vi "HFRR ADV v042.vi"() -> ()   [LabVIEW 2025] (continued)
            n2226 = call-poly <vilib>:"Mean.vi"("X"=w2445) -> ("mean"=→"КОФ2 4":dbl)  [unwired: 1 out]
            n2227 = call-poly <vilib>:"Mean.vi"("X"=w2508) -> ("mean"=→"КОФ3":dbl)  [unwired: 1 out]
            n2228 = call-poly <vilib>:"Mean.vi"("X"=w2503) -> ("mean"=→"CP3":dbl)  [unwired: 1 out]
            n2229 = Delete From Array(array=w2497, index=0) -> (array with subset deleted=w2424:dbl[])  [unwired: 1 in, 1 out]
            n2230 = Delete From Array(array=w2436, index=0) -> (array with subset deleted=w2423:dbl[])  [unwired: 1 in, 1 out]
            n2231 = Delete From Array(array=w2476, index=0) -> (array with subset deleted=w2447:dbl[])  [unwired: 1 in, 1 out]
            n2232 = Delete From Array(array=w2554, index=0) -> (array with subset deleted=w2509:dbl[])  [unwired: 1 in, 1 out]
            n2233 = Delete From Array(array=w2520, index=0) -> (array with subset deleted=w2505:dbl[])  [unwired: 1 in, 1 out]
            "array w/ subset deleted" <- w2505
            n2234 = Delete From Array(array=w2551, index=0) -> (array with subset deleted=w2552:dbl[])  [unwired: 1 in, 1 out]
            n2235 = call-poly <vilib>:"Mean.vi"("X"=w2447) -> ("mean"=→"КОФ2 2":dbl)  [unwired: 1 out]
            n2236 = call-poly <vilib>:"Mean.vi"("X"=w2509) -> ("mean"=→"КОФ1":dbl)  [unwired: 1 out]
            n2237 = Bundle "Bundle"(w2424, w2423) -> (w2429:cluster{dbl[], dbl[]})  [unwired: 1 in]
            n2238 = Bundle "Bundle"(w2424, w2552) -> (w2416:cluster{dbl[], dbl[]})  [unwired: 1 in]
            n2239 = Delete From Array(array=w2431, index=0) -> (array with subset deleted=w2419:dbl[])  [unwired: 1 in, 1 out]
            n2240 = Delete From Array(array=w2432, index=0) -> (array with subset deleted=w2421:dbl[])  [unwired: 1 in, 1 out]
            n2241 = Delete From Array(array=w2542, index=0) -> (array with subset deleted=w2543:dbl[])  [unwired: 1 in, 1 out]
            n2242 = Delete From Array(array=w2430, index=0) -> (array with subset deleted=w2417:dbl[])  [unwired: 1 in, 1 out]
            n2243 = Delete From Array(array=w2524, index=0) -> (array with subset deleted=w2525:dbl[])  [unwired: 1 in, 1 out]
            n2244 = Delete From Array(array=w2549, index=0) -> (array with subset deleted=w2455:dbl[])  [unwired: 1 in, 1 out]
            n2245 = Delete From Array(array=w2495, index=0) -> (array with subset deleted=w2451:dbl[])  [unwired: 1 in, 1 out]
            n2246 = Delete From Array(array=w2531, index=0) -> (array with subset deleted=w2453:dbl[])  [unwired: 1 in, 1 out]
            n2247 = Delete From Array(array=w2491, index=0) -> (array with subset deleted=w2449:dbl[])  [unwired: 1 in, 1 out]
            n2248 = Delete From Array(array=w2540, index=0) -> (array with subset deleted=w2454:dbl[])  [unwired: 1 in, 1 out]
            n2249 = Delete From Array(array=w2493, index=0) -> (array with subset deleted=w2450:dbl[])  [unwired: 1 in, 1 out]
            n2250 = Delete From Array(array=w2474, index=0) -> (array with subset deleted=w2446:dbl[])  [unwired: 1 in, 1 out]
            n2251 = Delete From Array(array=w2518, index=0) -> (array with subset deleted=w2504:dbl[])  [unwired: 1 in, 1 out]
            n2252 = Delete From Array(array=w2545, index=0) -> (array with subset deleted=w2506:dbl[])  [unwired: 1 in, 1 out]
            n2253 = Delete From Array(array=w2522, index=0) -> (array with subset deleted=w2452:dbl[])  [unwired: 1 in, 1 out]
            n2254 = Delete From Array(array=w2489, index=0) -> (array with subset deleted=w2448:dbl[])  [unwired: 1 in, 1 out]
            n2255 = Delete From Array(array=w2470, index=0) -> (array with subset deleted=w2444:dbl[])  [unwired: 1 in, 1 out]
            n2256 = Delete From Array(array=w2514, index=0) -> (array with subset deleted=w2502:dbl[])  [unwired: 1 in, 1 out]
            n2257 = Delete From Array(array=w2527, index=0) -> (array with subset deleted=w2507:dbl[])  [unwired: 1 in, 1 out]
            n2258 = Delete From Array(array=w2537, index=0) -> (array with subset deleted=w2420:dbl[])  [unwired: 1 in, 1 out]
            n2259 = Delete From Array(array=w2547, index=0) -> (array with subset deleted=w2422:dbl[])  [unwired: 1 in, 1 out]
            n2260 = Delete From Array(array=w2529, index=0) -> (array with subset deleted=w2418:dbl[])  [unwired: 1 in, 1 out]
            n2261 = Bundle "Bundle"(w2424, w2455) -> (w2442:cluster{dbl[], dbl[]})  [unwired: 1 in]
            n2262 = Bundle "Bundle"(w2424, w2509) -> (w2443:cluster{dbl[], dbl[]})  [unwired: 1 in]
            n2263 = Bundle "Bundle"(w2455, w2451) -> (w2457:cluster{dbl[], dbl[]})  [unwired: 1 in]
            n2264 = Bundle "Bundle"(w2420, w2419) -> (w2427:cluster{dbl[], dbl[]})  [unwired: 1 in]
            n2265 = Bundle "Bundle"(w2453, w2449) -> (w2459:cluster{dbl[], dbl[]})  [unwired: 1 in]
            n2266 = Bundle "Bundle"(w2420, w2453) -> (w2563:cluster{dbl[], dbl[]})  [unwired: 1 in]
            n2267 = Bundle "Bundle"(w2420, w2449) -> (w2487:cluster{dbl[], dbl[]})  [unwired: 1 in]
            n2268 = Bundle "Bundle"(w2420, w2508) -> (w2573:cluster{dbl[], dbl[]})  [unwired: 1 in]
            n2269 = Bundle "Bundle"(w2420, w2503) -> (w2511:cluster{dbl[], dbl[]})  [unwired: 1 in]
            n2270 = Bundle "Bundle"(w2420, w2534) -> (w2558:cluster{dbl[], dbl[]})  [unwired: 1 in]
            n2271 = Bundle "Bundle"(w2454, w2450) -> (w2458:cluster{dbl[], dbl[]})  [unwired: 1 in]
            n2272 = Bundle "Bundle"(w2422, w2421) -> (w2428:cluster{dbl[], dbl[]})  [unwired: 1 in]
            n2273 = Bundle "Bundle"(w2422, w2454) -> (w2565:cluster{dbl[], dbl[]})  [unwired: 1 in]
            n2274 = Bundle "Bundle"(w2422, w2450) -> (w2488:cluster{dbl[], dbl[]})  [unwired: 1 in]
            n2275 = Bundle "Bundle"(w2422, w2504) -> (w2512:cluster{dbl[], dbl[]})  [unwired: 1 in]
            n2276 = Bundle "Bundle"(w2422, w2506) -> (w2574:cluster{dbl[], dbl[]})  [unwired: 1 in]
            n2277 = Bundle "Bundle"(w2422, w2543) -> (w2556:cluster{dbl[], dbl[]})  [unwired: 1 in]
            n2278 = Bundle "Bundle"(w2452, w2448) -> (w2460:cluster{dbl[], dbl[]})  [unwired: 1 in]
            n2279 = Bundle "Bundle"(w2418, w2417) -> (w2426:cluster{dbl[], dbl[]})  [unwired: 1 in]
            n2280 = Bundle "Bundle"(w2418, w2452) -> (w2564:cluster{dbl[], dbl[]})  [unwired: 1 in]
            n2281 = Bundle "Bundle"(w2418, w2448) -> (w2486:cluster{dbl[], dbl[]})  [unwired: 1 in]
            n2282 = Bundle "Bundle"(w2418, w2502) -> (w2510:cluster{dbl[], dbl[]})  [unwired: 1 in]
            n2283 = Bundle "Bundle"(w2418, w2507) -> (w2572:cluster{dbl[], dbl[]})  [unwired: 1 in]
            n2284 = Bundle "Bundle"(w2418, w2525) -> (w2557:cluster{dbl[], dbl[]})  [unwired: 1 in]
            n2285 = call-poly <vilib>:"Mean.vi"("X"=w2505) -> ("mean"=→"CP1":dbl)  [unwired: 1 out]
            n2286 = call-poly <vilib>:"Mean.vi"("X"=w2446) -> ("mean"=→"КОФ2 3":dbl)  [unwired: 1 out]
            n2287 = call-poly <vilib>:"Mean.vi"("X"=w2504) -> ("mean"=→"CP2":dbl)  [unwired: 1 out]
            n2288 = call-poly <vilib>:"Mean.vi"("X"=w2506) -> ("mean"=→"КОФ2":dbl)  [unwired: 1 out]
            n2289 = call-poly <vilib>:"Mean.vi"("X"=w2444) -> ("mean"=→"КОФ2 5":dbl)  [unwired: 1 out]
            n2290 = call-poly <vilib>:"Mean.vi"("X"=w2502) -> ("mean"=→"CP4":dbl)  [unwired: 1 out]
            n2291 = call-poly <vilib>:"Mean.vi"("X"=w2507) -> ("mean"=→"КОФ4":dbl)  [unwired: 1 out]
            n2292 = Bundle "Bundle"(w2424, w2451) -> (w2415:cluster{dbl[], dbl[]})  [unwired: 1 in]
            n2293 = Bundle "Bundle"(w2424, w2505) -> (w2438:cluster{dbl[], dbl[]})  [unwired: 1 in]
            n2294 = Build Array "Build Array"(w2415, w2438) -> (w2441:cluster{dbl[], dbl[]}[])
            "XY Graph 17" <- w2441
            n2295 = Build Array "Build Array"(w2429, w2428, w2427, w2426) -> (→"Frequency ( Hz )":cluster{dbl[], dbl[]}[])
            n2296 = Build Array "Build Array"(w2457, w2458, w2459, w2460) -> (→"Air Temp ( °C ) vs Humidity ( % RH )":cluster{dbl[], dbl[]}[])
            n2297 = Build Array "Build Array"(w2442, w2565, w2563, w2564) -> (→"Air Temperature  ( °C )":cluster{dbl[], dbl[]}[])
            n2298 = Build Array "Build Array"(w2415, w2488, w2487, w2486) -> (→"Humidity ( %RH )":cluster{dbl[], dbl[]}[])
            n2299 = Build Array "Build Array"(w2443, w2574, w2573, w2572) -> (→"Coefficient Of Friction":cluster{dbl[], dbl[]}[])
            n2300 = Build Array "Build Array"(w2438, w2512, w2511, w2510) -> (→"Sample Temperature ( °C )":cluster{dbl[], dbl[]}[])
            n2301 = Build Array "Build Array"(w2416, w2556, w2558, w2557) -> (→"XY Graph 13":cluster{dbl[], dbl[]}[])
            n2302 = Bundle "Bundle"(w2424, w2447) -> (w2469:cluster{dbl[], dbl[]})  [unwired: 1 in]
            n2303 = Bundle "Bundle"(w2420, w2445) -> (w2467:cluster{dbl[], dbl[]})  [unwired: 1 in]
            n2304 = Bundle "Bundle"(w2422, w2446) -> (w2468:cluster{dbl[], dbl[]})  [unwired: 1 in]
            n2305 = Bundle "Bundle"(w2418, w2444) -> (w2466:cluster{dbl[], dbl[]})  [unwired: 1 in]
            n2306 = Build Array "Build Array"(w2469, w2468, w2467, w2466) -> (→"Stroke ( mm )":cluster{dbl[], dbl[]}[])
            n2307 = local write "XY Graph 16"(w2441) -> ()
          }
          frame #2 {
          }
          frame #3 {
            n2308 = local write "Numeric 8"(0 ("Numeric 8")) -> ()
            n2309 = local write "Numeric 11"(0 ("Numeric 11")) -> ()
            n2310 = local write "Numeric 12"(0 ("Numeric 12")) -> ()
            n2311 = local write "Numeric 13"(0 ("Numeric 13")) -> ()
            n2312 = property on="OPEN" class="Bool (strict)"("Visible"=TRUE) -> ()  [unwired: 2 in, 2 out]
            n2313 = local read "String Control 2"() -> (w2741:string)
            n2314 = local read "String Control 4"() -> (w2740:string)
            n2315 = local read "String Control 6"() -> (w2739:string)
            n2316 = local read "String Control 8"() -> (w2738:string)
            n2317 = Match Pattern(string=w2741, regular expression="Samples / cycle :- ") -> (after substring=w2755:string)  [unwired: 1 in, 3 out]
            n2318 = Match Pattern(string=w2741, regular expression="Frequency :- ") -> (after substring=w2774:string)  [unwired: 1 in, 3 out]
            n2319 = Match Pattern(string=w2740, regular expression="Samples / cycle :- ") -> (after substring=w2751:string)  [unwired: 1 in, 3 out]
            n2320 = Match Pattern(string=w2740, regular expression="Frequency :- ") -> (after substring=w2769:string)  [unwired: 1 in, 3 out]
            n2321 = Match Pattern(string=w2739, regular expression="Samples / cycle :- ") -> (after substring=w2747:string)  [unwired: 1 in, 3 out]
            n2322 = Match Pattern(string=w2739, regular expression="Frequency :- ") -> (after substring=w2764:string)  [unwired: 1 in, 3 out]
            n2323 = Match Pattern(string=w2738, regular expression="Samples / cycle :- ") -> (after substring=w2743:string)  [unwired: 1 in, 3 out]
            n2324 = Match Pattern(string=w2738, regular expression="Frequency :- ") -> (after substring=w2759:string)  [unwired: 1 in, 3 out]
            n2325 = String Subset(string=w2755, length (rest)=6 ("length (rest)")) -> (substring=w2757:string)  [unwired: 1 in]
            n2326 = String Subset(string=w2774, length (rest)=9 ("length (rest)")) -> (substring=w2776:string)  [unwired: 1 in]
            n2327 = String Subset(string=w2751, length (rest)=6 ("length (rest)")) -> (substring=w2753:string)  [unwired: 1 in]
            n2328 = String Subset(string=w2769, length (rest)=9 ("length (rest)")) -> (substring=w2771:string)  [unwired: 1 in]
            n2329 = String Subset(string=w2747, length (rest)=6 ("length (rest)")) -> (substring=w2749:string)  [unwired: 1 in]
            n2330 = String Subset(string=w2764, length (rest)=9 ("length (rest)")) -> (substring=w2766:string)  [unwired: 1 in]
            n2331 = String Subset(string=w2743, length (rest)=6 ("length (rest)")) -> (substring=w2745:string)  [unwired: 1 in]
            n2332 = String Subset(string=w2759, length (rest)=9 ("length (rest)")) -> (substring=w2761:string)  [unwired: 1 in]
            n2333 = Fract/Exp String To Number(string=w2757) -> (number=w2737:dbl)  [unwired: 3 in, 1 out]
            n2334 = Fract/Exp String To Number(string=w2776) -> (number=w2777:dbl)  [unwired: 3 in, 1 out]
            n2335 = Fract/Exp String To Number(string=w2753) -> (number=w2736:dbl)  [unwired: 3 in, 1 out]
            n2336 = Fract/Exp String To Number(string=w2771) -> (number=w2772:dbl)  [unwired: 3 in, 1 out]
            n2337 = Fract/Exp String To Number(string=w2749) -> (number=w2735:dbl)  [unwired: 3 in, 1 out]
            n2338 = Fract/Exp String To Number(string=w2766) -> (number=w2767:dbl)  [unwired: 3 in, 1 out]
            n2339 = Fract/Exp String To Number(string=w2745) -> (number=w2734:dbl)  [unwired: 3 in, 1 out]
            n2340 = Fract/Exp String To Number(string=w2761) -> (number=w2762:dbl)  [unwired: 3 in, 1 out]
            n2341 = local write "sample1"(w2737) -> ()
            n2342 = local write "freq1"(w2777) -> ()
            n2343 = local write "sample2"(w2736) -> ()
            n2344 = local write "freq2"(w2772) -> ()
            n2345 = local write "sample3"(w2735) -> ()
            n2346 = local write "freq3"(w2767) -> ()
            n2347 = local write "sample4"(w2734) -> ()
            n2348 = local write "freq 4"(w2762) -> ()
          }
        }
      }
    }
    n2349 = case shown="True" w2335 {
      selector: w2335 -> [_ w2354]
      frame False {
      }
      frame True {
        n2350 = Not(x=w2354) -> (.not. x?=w2350:bool)
        n2351 = local write "service 3"(w2350) -> ()
        n2352 = local write "OPEN 6"(w2350) -> ()
        n2353 = call <vilib>:"System Exec.vi"("wait until completion? (T)"=TRUE, "command line"="C:\\LAB-IQ\\Scar View.exe") -> ("error out"=→"error out 5":errorcluster)  [unwired: 6 in, 3 out]
      }
    }
    n2354 = case shown="\"Acquire\", Default" w2344 {
      frame "Acquire", Default {
        # "Elapsed time\ncof\nstroke\nAir temp\nTemp\nHumidity"
        n2355 = disable-structure shown="Disabled" {
          frame Disabled {
            n2356 = local read "Flag"() -> (w3053:dbl)
            n2357 = local read "RUN"() -> (w3050:bool)
            n2358 = Not(x=w3050) -> (.not. x?=w3049:bool)
            n2359 = Equal?(x=w3053, y=10.0) -> (x = y?=w3051:bool)
            n2360 = And(x=w3051, y=w3049) -> (x .and. y?=w3048:bool)
            n2361 = case shown="True" w3048 {
              frame False {
              }
              frame True {
                w3054 = FALSE ("Heater Button")
                n2362 = local write "Humidity"(w3054) -> ()
                n2363 = local write "Heater Button"(w3054) -> ()
              }
            }
          }
          frame Enabled {
          }
        }
        n2364 = disable-structure shown="Disabled" {
          frame Disabled {
            n2365 = case shown="True" {
              selector: _ -> [_ _]
              frame False {
              }
              frame True {
                w3099 = TRUE ("Heater")
                n2366 = local write "Humidity"(w3099) -> ()
                n2367 = local write "Heater Button"(w3099) -> ()
                n2368 = local read "TEST STANDARD"() -> (w3102:T3)
                n2369 = local read "TEST STANDARD"() -> (w3097:T3)
                n2370 = Equal?(x=w3102, y=enum16{"ASTM D6079", "ISO 12156", "Custom"}."ISO 12156" ("Test Standard")) -> (x = y?=w3100:bool)
                n2371 = Equal?(x=w3097, y=enum16{"ASTM D6079", "ISO 12156", "Custom"}."ASTM D6079" ("Test Standard")) -> (x = y?=w3096:bool)
                n2372 = case shown="True" w3100 {
                  frame False {
                  }
                  frame True {
                    n2373 = local write "airtempflg"(FALSE ("airtempflg")) -> ()
                    n2374 = local write item#-1(TRUE ("Heater")) -> ()
                  }
                }
                n2375 = case shown="True" w3096 {
                  frame False {
                  }
                  frame True {
                    n2376 = local write "airtempflg"(TRUE ("airtempflg")) -> ()
                    n2377 = local write item#-1(FALSE ("Heater")) -> ()
                  }
                }
              }
            }
          }
          frame Enabled {
          }
        }
        n2378 = stacked-sequence {
          frame #0 {
            n2379 = case shown="True" "RST FF" {
              frame False {
              }
              frame True {
                w3116 = 0.0 ("X Scale.Range:Maximum")
                n2380 = property on="Frictional Force ( N )" class="WFChart (strict)"("XScale.Maximum"=600.0 ("X Scale.Range:Maximum"), "XScale.Minimum"=w3116, "YScale.Maximum"=10.0 ("Y Scale.Range:Maximum"), "YScale.Minimum"=w3116) -> ()  [unwired: 2 in, 2 out]
              }
            }
          }
          frame #1 {
            n2381 = case shown="True" "RST TEMP" {
              frame False {
              }
              frame True {
                n2382 = property on="Temperature ( Deg C )" class="WFChart (strict)"("XScale.Minimum"=0.0 ("X Scale.Range:Minimum"), "XScale.Maximum"=600.0 ("X Scale.Range:Maximum"), "YScale.Minimum"=0.0 ("Y Scale.Range:Minimum"), "YScale.Maximum"=100.0 ("Y Scale.Range:Maximum")) -> ()  [unwired: 2 in, 2 out]
              }
            }
          }
          frame #2 {
            n2383 = case shown="True" "RSTCOF" {
              frame False {
              }
              frame True {
                n2384 = property on="Coefficient of Friction" class="WFChart (strict)"("XScale.Minimum"=0.0 ("X Scale.Range:Minimum"), "XScale.Maximum"=600.0 ("X Scale.Range:Maximum"), "YScale.Maximum"=1.0 ("X Scale.Range:Minimum"), "YScale.Minimum"=0.0 ("X Scale.Range:Minimum")) -> ()  [unwired: 2 in, 2 out]
              }
            }
          }
          frame #3 {
            n2385 = case shown="True" "RSTCOF 2" {
              frame False {
              }
              frame True {
                (unwired) 100.0 ("Y Scale.Range:Maximum")
                (unwired) 0.0 ("Y Scale.Range:Minimum")
                (unwired) 600.0 ("X Scale.Range:Maximum")
                (unwired) 0.0 ("X Scale.Range:Minimum")
              }
            }
          }
          frame #4 {
            n2386 = case shown="True" "RSTCOF 3" {
              frame False {
              }
              frame True {
                n2387 = property on="Electrical Contact Resistance ( % )" class="WFChart (strict)"("XScale.Minimum"=0.0 ("X Scale.Range:Minimum"), "XScale.Maximum"=600.0 ("X Scale.Range:Maximum"), "YScale.Minimum"=0.0 ("Y Scale.Range:Minimum"), "YScale.Maximum"=100.0 ("Y Scale.Range:Maximum")) -> ()  [unwired: 2 in, 2 out]
              }
            }
          }
        }
        n2388 = local read "RUN"() -> (w3043:bool)
        n2389 = case shown="False" w3043 {
          frame False {
          }
          frame True {
          }
        }
        n2390 = local read "RUN"() -> (w3047:bool)
        n2391 = case shown="False" w3047 {
          tunnel: [FALSE ("TEST RUNNING") TRUE ("TEST RUNNING")] -> w3046
          frame False {
            w3135 = 0.0 ("Flag")
            n2392 = local write "Elapsed time"(0.0 ("elapsedtime")) -> ()
            n2393 = local write "Time Remaining"(w3135) -> ()
            n2394 = local write "Flag"(w3135) -> ()
            n2395 = local write "Remaining Time"(w3135) -> ()
          }
          frame True {
            n2396 = local write "Flag"(10.0 ("Flag")) -> ()
          }
        }
        n2397 = local read "AIR TEMP"() -> (w3041:dbl)
        n2398 = Greater Or Equal?(x=w3041, y=15.0) -> (x >= y?=w3042:bool)
        "powstat" <- w3042
        n2399 = case shown="True" "Save & Continue" {
          frame False {
          }
          frame True {
            n2400 = local read "USER ID"() -> (w3439:string)
            n2401 = local read "FILE"() -> (w3447:string)
            n2402 = String Length(string=w3447) -> (length=w3445:i32)
            n2403 = String Length(string=w3439) -> (length=w3442:i32)
            n2404 = Greater?(x=w3445, y=0) -> (0:w3444:bool)
            n2405 = Greater?(x=w3442, y=0) -> (0:w3441:bool)
            n2406 = And(x=w3444, y=w3441) -> (x .and. y?=w3440:bool)
            n2407 = case shown="True" w3440 {
              frame False {
                n2408 = stacked-sequence {
                  frame #0 {
                    n2409 = One Button Dialog(message="Please Enter a File Name and Operator ID to save data !", button name ("OK")="Ok") -> ()  [unwired: 1 out]
                  }
                  frame #1 {
                    n2410 = local write "Save & Continue"(FALSE ("OK Button")) -> ()
                  }
                }
                n2411 = local write "Save & Continue"(FALSE ("OK Button")) -> ()
              }
              frame True {
                n2412 = stacked-sequence {
                  frame #0 {
                    n2413 = local read "FILE"() -> (w3453:string)
                    n2414 = call "file check.vi"("file name in"=w3453) -> ("file name out"=w3452:string)  [unwired: 9 in, 1 out]
                    n2415 = call <vilib>:"Application Directory.vi"() -> ("Application Directory"=w3463:path)
                    n2416 = Build Path(base path=w3463, name or relative path="data") -> (appended path=w3462:path)
                    n2417 = call <vilib>:"Trim Whitespace.vi"("string"=w3452) -> ("trimmed string"=w3460:string)  [unwired: 1 in]
                    n2418 = call <vilib>:"Trim Whitespace.vi"("string"=w3452) -> ("trimmed string"=w3461:string)  [unwired: 1 in]
                    n2419 = List Folder(path=w3462) -> (folder names=w3458:string[])  [unwired: 3 in, 3 out]
                    n2420 = Match Pattern(string=w3460, regular expression="_(") -> (before substring=w3457:string)  [unwired: 1 in, 3 out]
                    n2421 = for {
                      tunnel: w3458 -> [w3472] mode=indexing
                      tunnel: w3457 -> [w3470]
                      shift-right: [w3468] -> w3455
                      shift-left: bool[] [] -> [w3469]
                      n2422 = Match Pattern(string=w3472, regular expression="_(") -> (before substring=w3471:string)  [unwired: 1 in, 3 out]
                      n2423 = Equal?(x=w3471, y=w3470) -> (x = y?=w3467:bool)
                      n2424 = case shown="True" w3467 {
                        tunnel: w3467 -> [_ w3475]
                        tunnel: w3469 -> [w3474 w3477]
                        tunnel: [w3474 w3476] -> w3468
                        frame False {
                        }
                        frame True {
                          n2425 = Insert Into Array(array=w3477, new element=w3475) -> (w3476:bool[])  [unwired: 1 in]
                        }
                      }
                    }
                    n2426 = Equal?(x=w3458, y=w3457) -> (x = y?=w3466:bool[])
                    n2427 = Or Array Elements(Boolean array=w3466) -> (logical OR=w3465:bool)
                    n2428 = Array Size(array=w3455) -> (size(s)=w3454:i32)
                    n2429 = case shown="True" w3465 {
                      tunnel: w3461 -> [_ w3485]
                      tunnel: w3454 -> [_ w3478]
                      frame False {
                      }
                      frame True {
                        n2430 = Number To Decimal String(number=w3478) -> (decimal integer string=w3481:string)  [unwired: 1 in]
                        n2431 = Search/Split String(string=w3485, search string/char (-)="_(" ("regular expression")) -> (substring before match=w3483:string)  [unwired: 1 in, 2 out]
                        n2432 = Concatenate Strings(w3483, "_(" ("regular expression"), w3481, ")" ("regular expression")) -> (w3479:string)
                        n2433 = local write "FILE"(w3479) -> ()
                      }
                    }
                  }
                  frame #1 {
                    w3488 = 0.0
                    w3501 = cluster{"y":dbl, dbl, "y":dbl}[] [] ("History Data")
                    w3502 = FALSE ("Heater Button")
                    (unwired) ")!" ("string")
                    (unwired) ")" ("string")
                    w3500 = dbl[] [] ("History Data")
                    w3506 = "\r"
                    # "C:\\WinDucom\\Data\\"
                    # "C:\\LAB-IQ-NXT\\data"
                    n2434 = local write "Humidity ( %RH )"(w3488) -> ()
                    n2435 = local write "Frequency ( Hz )"(w3488) -> ()
                    n2436 = local write "Stroke 3"(w3488) -> ()
                    n2437 = local write "speedop"(0.0 ("PIDclk 2")) -> ()
                    n2438 = local write "Set Temp 2"(65.0 ("Set Temp 2")) -> ()
                    n2439 = local write "AIR TEMP"(w3488) -> ()
                    n2440 = local write "clk"(0.0 ("clk")) -> ()
                    n2441 = local write "Stroke 4"(w3488) -> ()
                    n2442 = local write "COF 2"(w3488) -> ()
                    n2443 = local write "TEMP"(w3488) -> ()
                    n2444 = local write "ecr 3"(w3488) -> ()
                    n2445 = local write "FF 3"(w3488) -> ()
                    n2446 = local write "FF 2"(w3488) -> ()
                    n2447 = property on="Coefficient of Friction" class="WFChart (strict)"("History Data"=w3500) -> ()  [unwired: 2 in, 2 out]
                    n2448 = property on="Coefficient of Friction" class="WFChart (strict)"("History Data"=w3500) -> ()  [unwired: 2 in, 2 out]
                    n2449 = property on="Frictional Force ( N )" class="WFChart (strict)"("History Data"=w3500) -> ()  [unwired: 2 in, 2 out]
                    n2450 = property on="Electrical Contact Resistance ( % )" class="WFChart (strict)"("History Data"=w3500) -> ()  [unwired: 2 in, 2 out]
                    n2451 = property on="Electrical Contact Resistance ( % )" class="WFChart (strict)"("History Data"=w3500) -> ()  [unwired: 2 in, 2 out]
                    n2452 = property on="Temperature ( Deg C )" class="WFChart (strict)"("History Data"=w3500) -> ()  [unwired: 2 in, 2 out]
                    n2453 = property on="Frictional Force ( N )" class="WFChart (strict)"("History Data"=w3500) -> ()  [unwired: 2 in, 2 out]
                    n2454 = property on="Coefficient of Friction" class="WFChart (strict)"("History Data"=w3500) -> ()  [unwired: 2 in, 2 out]
                    n2455 = property on="Frictional Force ( N )" class="WFChart (strict)"("History Data"=w3500) -> ()  [unwired: 2 in, 2 out]
                    n2456 = property on="Electrical Contact Resistance ( % )" class="WFChart (strict)"("History Data"=w3500) -> ()  [unwired: 2 in, 2 out]
                    n2457 = property on="Temperature ( Deg C )" class="WFChart (strict)"("History Data"=w3500) -> ()  [unwired: 2 in, 2 out]
                    n2458 = property on="Stroke ( mm )" class="WFChart (strict)"("History Data"=w3501) -> ()  [unwired: 2 in, 2 out]
                    n2459 = property on="Stroke ( mm )" class="WFChart (strict)"("History Data"=w3501) -> ()  [unwired: 2 in, 2 out]
                    n2460 = local write "Humidity"(w3502) -> ()
                    n2461 = local write "Heater Button"(w3502) -> ()
                    n2462 = local read "FILE"() -> (w3496:string)
                    n2463 = disable-structure shown="Enabled" {
                      disable-tunnel: [w3540 _] -> w3487
                      frame Enabled {
                        n2464 = local read "NORMAL LOAD"() -> (w3540:dbl)
                      }
                      frame Disabled {
                      }
                    }
                    n2465 = call "file check.vi"("file name in"=w3496) -> ("error out"=w3499:errorcluster, "file name out"=w3493:string)  [unwired: 9 in]
                    n2466 = call "FILE PATH CREATION.vi"("error in"=w3499, "FILE NAME :"=w3493) -> ("FILE OUT"=w3492:path)  [unwired: 8 in, 1 out]
                    n2467 = Concatenate Strings(w3493, ".dgf" ("Substring")) -> (w3498:string)
                    n2468 = Concatenate Strings(w3493, ".duf" ("Substring")) -> (w3494:string)
                    n2469 = Multiply(x=w3487, y=1.0) -> (x*y=w3519:dbl)
                    n2470 = Build Path(base path=w3492, name or relative path=w3498) -> (appended path=w3491:path)
                    n2471 = Build Path(base path=w3492, name or relative path=w3494) -> (appended path=w3490:path)
                    n2472 = Number To Fractional String(number=w3519, width (-)=i16 5, precision (6)=i16 2) -> (F-format string=w3527:string)  [unwired: 1 in]
                    n2473 = local read "tested by"() -> (w3486:string)
                    n2474 = local read "Fuel Discription :"() -> (w3515:string)
                    n2475 = local read "Batch Ref Num :"() -> (w3504:string)
                    n2476 = Get Date/Time String(date format (0)=enum16{"short", "long", "abbreviated"}."short") -> (date string=w3538:string, time string=w3535:string)  [unwired: 2 in]
                    n2477 = local read "Remarks :"() -> (w3514:string)
                    n2478 = Concatenate Strings("Load :- " ("Substring"), w3527, " grams ," ("Substring")) -> (w3526:string)
                    n2479 = local read "String 41"() -> (w3507:string)
                    n2480 = Concatenate Strings(w3515) -> (w3516:string)
                    n2481 = Concatenate Strings(w3504) -> (w3503:string)
                    n2482 = Concatenate Strings(w3486) -> (w3510:string)
                    n2483 = Concatenate Strings("(" ("Substring"), w3538, ")" ("Substring"), w3535) -> (w3509:string)
                    "concatenated string" <- w3509
                    n2484 = Concatenate Strings(w3514, "," ("string")) -> (w3513:string)
                    n2485 = Concatenate Strings("  TIME;      COF;       STROKE;     AIR TEMP;  TEMP;  HUMIDITY;  ECR; PID-OUT; FREQUENCY" ("Substring"), "\r") -> (w3522:string)
                    n2486 = Concatenate Strings(w3507, w3506, "Fuel Discription :-" ("Substring"), w3516, w3506, w3526, w3506, "Batch Ref Num :-" ("Substring"), w3503, w3506, " Remarks :- " ("Substring"), w3513, w3506, " Date :- " ("Substring"), w3509, w3506, "Tested By :-" ("Substring"), w3510) -> (w3520:string)
                    "REMARKS" <- w3520
                    n2487 = call <vilib>:"Write Characters To File.vi"("append to file? (new file:F)"=FALSE, "character string"=w3522, "file path (dialog if empty)"=w3491) -> ()  [unwired: 2 in, 1 out]
                    n2488 = call <vilib>:"Write Characters To File.vi"("append to file? (new file:F)"=FALSE, "character string"=w3520, "file path (dialog if empty)"=w3490) -> ()  [unwired: 2 in, 1 out]
                  }
                  frame #2 {
                    n2489 = local write "Cycles elapsed"(0 ("Cycles elapsed")) -> ()
                    n2490 = local write "cyclecount"(0 ("cyclecount")) -> ()
                    n2491 = local write "Save & Continue"(FALSE ("OK")) -> ()
                    n2492 = local write "autostrtflg"(TRUE ("autostrtflg")) -> ()
                    n2493 = local write "Save"(FALSE ("Save")) -> ()
                    n2494 = Get Date/Time In Seconds() -> (seconds since 1Jan1904=w3545:timestamp)
                    n2495 = To Double Precision Float(number=w3545) -> (double precision float=w3544:dbl)
                    n2496 = local write "acq timer"(w3544) -> ()
                    n2497 = One Button Dialog(message="Please ensure sample is mounted properly and machine is ready in all aspects for testing !", button name ("OK")="Ok") -> ()  [unwired: 1 out]
                  }
                  frame #3 {
                    n2498 = stacked-sequence {
                      frame #0 {
                        n2499 = local write "Main Dashboard Buttons"(T1."Dashboard" ("Main Dashboard Buttons")) -> ()
                        n2500 = local write "Main Tab"(T2."Acquire" ("Main Tab")) -> ()
                      }
                      frame #1 {
                        n2501 = local write "EVENT LOG"("" ("EVENT LOG")) -> ()
                      }
                      frame #2 {
                        n2502 = Wait (ms)(milliseconds to wait=u32 50) -> ()  [unwired: 1 out]
                      }
                      frame #3 {
                        n2503 = disable-structure shown="Disabled" {
                          frame Disabled {
                            n2504 = local read "EVENT LOG"() -> (w3557:string)
                            n2505 = call "Event Log.vi"("Content"="Test Details", "EVENT LOG"=w3557) -> ("EVENT LOG"=w3556:string)  [unwired: 8 in, 1 out]
                            n2506 = local write "EVENT LOG"(w3556) -> ()
                          }
                          frame Enabled {
                          }
                        }
                      }
                      frame #4 {
                        n2507 = Wait (ms)(milliseconds to wait=u32 50) -> ()  [unwired: 1 out]
                      }
                      frame #5 {
                        n2508 = local read "FILE"() -> (w3559:string)
                        n2509 = Concatenate Strings("File Name :" ("Content"), w3559) -> (w3560:string)
                        n2510 = local read "EVENT LOG"() -> (w3563:string)
                        n2511 = call "Event Log.vi"("Content"=w3560, "EVENT LOG"=w3563) -> ("EVENT LOG"=w3562:string)  [unwired: 8 in, 1 out]
                        n2512 = local write "EVENT LOG"(w3562) -> ()
                      }
                      frame #6 {
                        n2513 = Wait (ms)(milliseconds to wait=u32 50) -> ()  [unwired: 1 out]
                      }
                      frame #7 {
                        n2514 = local read "Batch Ref Num :"() -> (w3565:string)
                        n2515 = Concatenate Strings("Batch Ref No :" ("Content"), w3565) -> (w3566:string)
                        n2516 = local read "EVENT LOG"() -> (w3569:string)
                        n2517 = call "Event Log.vi"("Content"=w3566, "EVENT LOG"=w3569) -> ("EVENT LOG"=w3568:string)  [unwired: 8 in, 1 out]
                        n2518 = local write "EVENT LOG"(w3568) -> ()
                      }
                      frame #8 {
                        n2519 = Wait (ms)(milliseconds to wait=u32 50) -> ()  [unwired: 1 out]
                      }
                      frame #9 {
                        n2520 = local read "tested by"() -> (w3571:string)
                        n2521 = Concatenate Strings("Tested By :" ("Content"), w3571) -> (w3572:string)
                        n2522 = local read "EVENT LOG"() -> (w3575:string)
                        n2523 = call "Event Log.vi"("Content"=w3572, "EVENT LOG"=w3575) -> ("EVENT LOG"=w3574:string)  [unwired: 8 in, 1 out]
                        n2524 = local write "EVENT LOG"(w3574) -> ()
                      }
                      frame #10 {
                        n2525 = Wait (ms)(milliseconds to wait=u32 50) -> ()  [unwired: 1 out]
                      }
                      frame #11 {
                        n2526 = local read "TEST STANDARD"() -> (w3578:T3)
                        n2527 = case shown="\"ASTM D6079\", Default" w3578 {
                          tunnel: ["ASTM D6079" "ISO 12156" "CEC F-096-A-06" "Custom"] -> w3577
                          frame "ASTM D6079", Default {
                          }
                          frame "ISO 12156" {
                          }
                          frame "CEC F-096-A-06" {
                          }
                          frame "Custom" {
                          }
                        }
                        n2528 = Concatenate Strings("Test Standard :" ("Content"), w3577) -> (w3579:string)
                        n2529 = local read "EVENT LOG"() -> (w3582:string)
                        n2530 = call "Event Log.vi"("Content"=w3579, "EVENT LOG"=w3582) -> ("EVENT LOG"=w3581:string)  [unwired: 8 in, 1 out]
                        n2531 = local write "EVENT LOG"(w3581) -> ()
                      }
                      frame #12 {
                        n2532 = Wait (ms)(milliseconds to wait=u32 50) -> ()  [unwired: 1 out]
                      }
                      frame #13 {
                        n2533 = local read "Fuel Discription :"() -> (w3588:string)
                        n2534 = Concatenate Strings("Fuel Description :" ("Content"), w3588) -> (w3589:string)
                        n2535 = local read "EVENT LOG"() -> (w3592:string)
                        n2536 = call "Event Log.vi"("Content"=w3589, "EVENT LOG"=w3592) -> ("EVENT LOG"=w3591:string)  [unwired: 8 in, 1 out]
                        n2537 = local write "EVENT LOG"(w3591) -> ()
                      }
                      frame #14 {
                        n2538 = Wait (ms)(milliseconds to wait=u32 50) -> ()  [unwired: 1 out]
                      }
                      frame #15 {
                        n2539 = local read "Remarks :"() -> (w3594:string)
                        n2540 = Concatenate Strings("Remarks :" ("Content"), w3594) -> (w3595:string)
                        n2541 = local read "EVENT LOG"() -> (w3598:string)
                        n2542 = call "Event Log.vi"("Content"=w3595, "EVENT LOG"=w3598) -> ("EVENT LOG"=w3597:string)  [unwired: 8 in, 1 out]
                        n2543 = local write "EVENT LOG"(w3597) -> ()
                      }
                      frame #16 {
                        n2544 = Wait (ms)(milliseconds to wait=u32 50) -> ()  [unwired: 1 out]
                      }
                      frame #17 {
                        n2545 = local read "USER ID"() -> (w3600:string)
                        n2546 = Concatenate Strings("Operator ID :" ("Content"), w3600) -> (w3602:string)
                        n2547 = local read "EVENT LOG"() -> (w3604:string)
                        n2548 = call "Event Log.vi"("Content"=w3602, "EVENT LOG"=w3604) -> ("EVENT LOG"=w3603:string)  [unwired: 8 in, 1 out]
                        n2549 = local write "EVENT LOG"(w3603) -> ()
                      }
                      frame #18 {
                        n2550 = Wait (ms)(milliseconds to wait=u32 50) -> ()  [unwired: 1 out]
                      }
                      frame #19 {
                        n2551 = disable-structure shown="Disabled" {
                          frame Disabled {
                            n2552 = local read "EVENT LOG"() -> (w3608:string)
                            n2553 = call "Event Log.vi"("Content"="Test Parameter", "EVENT LOG"=w3608) -> ("EVENT LOG"=w3607:string)  [unwired: 8 in, 1 out]
                            n2554 = local write "EVENT LOG"(w3607) -> ()
                          }
                          frame Enabled {
                          }
                        }
                      }
                      frame #20 {
                        n2555 = Wait (ms)(milliseconds to wait=u32 50) -> ()  [unwired: 1 out]
                      }
                      frame #21 {
                        n2556 = local read "Set Hz"() -> (w3612:dbl)
                        n2557 = Number To Fractional String(number=w3612, precision (6)=i16 2) -> (F-format string=w3611:string)  [unwired: 2 in]
                        n2558 = Concatenate Strings("Set Frequency [Hz] :" ("Content"), w3611) -> (w3614:string)
                        n2559 = local read "EVENT LOG"() -> (w3616:string)
                        n2560 = call "Event Log.vi"("Content"=w3614, "EVENT LOG"=w3616) -> ("EVENT LOG"=w3615:string)  [unwired: 8 in, 1 out]
                        n2561 = local write "EVENT LOG"(w3615) -> ()
                      }
                      frame #22 {
                        n2562 = Wait (ms)(milliseconds to wait=u32 50) -> ()  [unwired: 1 out]
                      }
                      frame #23 {
                        n2563 = local read "NORMAL LOAD"() -> (w3619:dbl)
                        n2564 = Number To Fractional String(number=w3619, precision (6)=i16 2) -> (F-format string=w3620:string)  [unwired: 2 in]
                        n2565 = Concatenate Strings("Applied Load [grams] :" ("Content"), w3620) -> (w3622:string)
                        n2566 = local read "EVENT LOG"() -> (w3624:string)
                        n2567 = call "Event Log.vi"("Content"=w3622, "EVENT LOG"=w3624) -> ("EVENT LOG"=w3623:string)  [unwired: 8 in, 1 out]
                        n2568 = local write "EVENT LOG"(w3623) -> ()
                      }
                      frame #24 {
                        n2569 = Wait (ms)(milliseconds to wait=u32 50) -> ()  [unwired: 1 out]
                      }
                      frame #25 {
                        n2570 = local read "Set Strk"() -> (w3627:dbl)
                        n2571 = Number To Fractional String(number=w3627, precision (6)=i16 2) -> (F-format string=w3628:string)  [unwired: 2 in]
                        n2572 = Concatenate Strings("Set Stroke [mm] :" ("Content"), w3628) -> (w3630:string)
                        n2573 = local read "EVENT LOG"() -> (w3632:string)
                        n2574 = call "Event Log.vi"("Content"=w3630, "EVENT LOG"=w3632) -> ("EVENT LOG"=w3631:string)  [unwired: 8 in, 1 out]
                        n2575 = local write "EVENT LOG"(w3631) -> ()
                      }
                      frame #26 {
                        n2576 = Wait (ms)(milliseconds to wait=u32 50) -> ()  [unwired: 1 out]
                      }
                      frame #27 {
                        n2577 = local read "Set Temp"() -> (w3635:dbl)
                        n2578 = Number To Fractional String(number=w3635, precision (6)=i16 2) -> (F-format string=w3636:string)  [unwired: 2 in]
                        n2579 = Concatenate Strings("Set Temperature [deg C] :" ("Content"), w3636) -> (w3638:string)
                        n2580 = local read "EVENT LOG"() -> (w3640:string)
                        n2581 = call "Event Log.vi"("Content"=w3638, "EVENT LOG"=w3640) -> ("EVENT LOG"=w3639:string)  [unwired: 8 in, 1 out]
                        n2582 = local write "EVENT LOG"(w3639) -> ()
                      }
                      frame #28 {
                        n2583 = Wait (ms)(milliseconds to wait=u32 50) -> ()  [unwired: 1 out]
                      }
                      frame #29 {
                        n2584 = local read "Set Rh"() -> (w3643:dbl)
                        n2585 = Number To Fractional String(number=w3643, precision (6)=i16 2) -> (F-format string=w3644:string)  [unwired: 2 in]
                        n2586 = Concatenate Strings("Set Humidity [%RH] :" ("Content"), w3644) -> (w3646:string)
                        n2587 = local read "EVENT LOG"() -> (w3648:string)
                        n2588 = call "Event Log.vi"("Content"=w3646, "EVENT LOG"=w3648) -> ("EVENT LOG"=w3647:string)  [unwired: 8 in, 1 out]
                        n2589 = local write "EVENT LOG"(w3647) -> ()
                      }
                      frame #30 {
                        n2590 = Wait (ms)(milliseconds to wait=u32 50) -> ()  [unwired: 1 out]
                      }
                      frame #31 {
                        n2591 = local read "test time"() -> (w3651:dbl)
                        n2592 = Number To Fractional String(number=w3651, precision (6)=i16 1) -> (F-format string=w3652:string)  [unwired: 2 in]
                        n2593 = Concatenate Strings("Test Duration [mins] :" ("Content"), w3652) -> (w3654:string)
                        n2594 = local read "EVENT LOG"() -> (w3656:string)
                        n2595 = call "Event Log.vi"("Content"=w3654, "EVENT LOG"=w3656) -> ("EVENT LOG"=w3655:string)  [unwired: 8 in, 1 out]
                        n2596 = local write "EVENT LOG"(w3655) -> ()
                      }
                      frame #32 {
                        w3657 = dbl[] [] ("History Data")
                        w3658 = cluster{"y":dbl, dbl, "y":dbl}[] [] ("History Data")
                        w3659 = FALSE ("Visible")
                        n2597 = property on="Stroke ( mm )" class="WFChart (strict)"("History Data"=w3658) -> ()  [unwired: 2 in, 2 out]
                        n2598 = property on="Temperature ( Deg C )" class="WFChart (strict)"("History Data"=w3657) -> ()  [unwired: 2 in, 2 out]
                        n2599 = property on="Electrical Contact Resistance ( % )" class="WFChart (strict)"("History Data"=w3657) -> ()  [unwired: 2 in, 2 out]
                        n2600 = property on="Coefficient of Friction" class="WFChart (strict)"("History Data"=w3657) -> ()  [unwired: 2 in, 2 out]
                        n2601 = property on="Frictional Force ( N )" class="WFChart (strict)"("History Data"=w3657) -> ()  [unwired: 2 in, 2 out]
                        n2602 = property on="Coefficient of Friction" class="WFChart (strict)"("History Data"=w3657) -> ()  [unwired: 2 in, 2 out]
                        n2603 = property on="Frictional Force ( N )" class="WFChart (strict)"("History Data"=w3657) -> ()  [unwired: 2 in, 2 out]
                        n2604 = property on="Electrical Contact Resistance ( % )" class="WFChart (strict)"("History Data"=w3657) -> ()  [unwired: 2 in, 2 out]
                        n2605 = property on="Stroke ( mm )" class="WFChart (strict)"("History Data"=w3658) -> ()  [unwired: 2 in, 2 out]
                        n2606 = property on="Temperature ( Deg C )" class="WFChart (strict)"("History Data"=w3657) -> ()  [unwired: 2 in, 2 out]
                        n2607 = property on="Service Password Log" class="Str"("Visible"=w3659) -> ()  [unwired: 2 in, 2 out]
                        n2608 = property on="Password 3" class="Clust (strict)"("Visible"=w3659) -> ()  [unwired: 2 in, 2 out]
                      }
                    }
                    "TEST FILE NAM,E SAVED" <- TRUE ("TEST FILE NAM,E SAVED")
                  }
                }
              }
            }
          }
        }
        n2609 = local write "Test \nStatus"(w3046) -> ()
        n2610 = local write "Save"(w3046) -> ()
        n2611 = local read "Main Tab"() -> (w3040:T2)
        n2612 = case shown="True" w3043 {
          frame False {
            n2613 = local read "Rt 3"() -> (w3107:bool)
            n2614 = case shown="True" w3107 {
              frame False {
              }
              frame True {
                n2615 = local write "Rt 3"(FALSE ("Rt 3")) -> ()
              }
            }
            "Rt" <- TRUE ("Rt")
            "Rt 2" <- FALSE ("Rt")
          }
          frame True {
            n2616 = local read "Rt"() -> (w3113:bool)
            n2617 = local write "Rt 2"(TRUE ("Rt 2")) -> ()
            n2618 = case shown="True" w3113 {
              frame False {
              }
              frame True {
                n2619 = local write "Rt"(FALSE ("Rt")) -> ()
              }
            }
            "Rt 3" <- TRUE ("Rt 3")
          }
        }
        n2620 = case shown="\"Acquire\"" w3040 {
          tunnel: w3042 -> [_ w3142]
          frame Default {
            w3141 = 0.0 ("output")
            n2621 = local write "PID-out"(w3141) -> ()
            n2622 = local write "Frequency ( Hz )"(w3141) -> ()
            n2623 = local write "STROKE Initialize"(TRUE ("STROKE Initialize")) -> ()
          }
          frame "Acquire" {
            n2624 = stacked-sequence {
              frame #0 {
                n2625 = local read "Auto Start Test"() -> (w3144:bool)
                n2626 = case shown="True" w3144 {
                  tunnel: "RUN" -> [w3165 w3168]
                  tunnel: [w3165 w3167] -> w3145
                  frame False {
                  }
                  frame True {
                    n2627 = local read "Auto Start Temp"() -> (w3166:bool)
                    n2628 = Or(x=w3168, y=w3166) -> (x .or. y?=w3167:bool)
                  }
                }
                n2629 = local read "clk"() -> (w3164:dbl)
                n2630 = local read "Save"() -> (w3160:bool)
                n2631 = Equal?(x=w3164, y=0.0) -> (x = y?=w3161:bool)
                n2632 = And(x=w3161, y=w3160) -> (x .and. y?=w3162:bool)
                n2633 = Not(x="Engage") -> (.not. x?=w3151:bool)
                n2634 = case shown="False" w3145 {
                  tunnel: [0.0 w3192] -> w3147
                  frame False {
                    (unwired) TRUE ("Visible")
                    n2635 = local read "Auto Start Test"() -> (w3172:bool)
                    n2636 = local write "Start Time"(TRUE ("Start Time")) -> ()
                    n2637 = property on="Stroke 2" class="DigNum (strict)"("Visible"=FALSE) -> ()  [unwired: 2 in, 2 out]
                    n2638 = case shown="False" w3172 {
                      frame False {
                        n2639 = property on="Heater Button" class="Bool (strict)"("DisabledEnum"=T19."Enabled" ("Disabled")) -> ()  [unwired: 2 in, 2 out]
                        n2640 = property on="Humidity" class="Bool (strict)"("DisabledEnum"=T19."Enabled" ("Disabled")) -> ()  [unwired: 2 in, 2 out]
                      }
                      frame True {
                      }
                    }
                    n2641 = case shown="False" "TestCompFlg" {
                      frame False {
                        n2642 = local read "StartFlg"() -> (w3180:bool)
                        n2643 = case shown="True" w3180 {
                          frame False {
                          }
                          frame True {
                            n2644 = stacked-sequence {
                              frame #0 {
                                n2645 = local read "EVENT LOG"() -> (w3184:string)
                                n2646 = call "Event Log.vi"("Content"="Test was interrupted", "EVENT LOG"=w3184) -> ("EVENT LOG"=w3185:string)  [unwired: 8 in, 1 out]
                                n2647 = local write "EVENT LOG"(w3185) -> ()
                                n2648 = property on="RUN" class="Bool (strict)"("Visible"=TRUE) -> ()  [unwired: 2 in, 2 out]
                                n2649 = property on="Auto Start Test" class="Bool (strict)"("Visible"=TRUE) -> ()  [unwired: 2 in, 2 out]
                              }
                              frame #1 {
                                w3188 = FALSE ("StartFlg")
                                n2650 = property on="Heater Button" class="Bool (strict)"("Val(Sgnl)"=FALSE ("Value (Signaling)")) -> ()  [unwired: 2 in, 2 out]
                                n2651 = local write "Heater Button"(w3188) -> ()
                                n2652 = local write "StartFlg"(w3188) -> ()
                                n2653 = local write "Humidity"(w3188) -> ()
                                n2654 = local write "Humidity 2"(TRUE ("Humidity")) -> ()
                              }
                              frame #2 {
                                n2655 = local write "Due Write"("VC;0" ("Command")) -> ()
                              }
                              frame #3 {
                                n2656 = Wait (ms)(milliseconds to wait=u32 1500) -> ()  [unwired: 1 out]
                              }
                              frame #4 {
                                n2657 = local write "Due Write"("HE;0" ("Command")) -> ()
                              }
                            }
                          }
                        }
                      }
                      frame True {
                      }
                    }
                    n2658 = local write "String 14"("Test will autostart once parameters reach the set value." ("String 14")) -> ()
                  }
                  frame True {
                    (unwired) FALSE ("Visible")
                    n2659 = property on="Stroke 2" class="DigNum (strict)"("Visible"=TRUE) -> ()  [unwired: 2 in, 2 out]
                    n2660 = property on="STOP 2" class="Bool (strict)"("Disabled"=u8 2) -> ()  [unwired: 2 in, 2 out]
                    n2661 = local write "String 14"(" Running....." ("String 14")) -> ()
                    n2662 = property on="Heater Button" class="Bool (strict)"("DisabledEnum"=T19."Disabled and Grayed Out" ("Disabled")) -> ()  [unwired: 2 in, 2 out]
                    n2663 = property on="Humidity" class="Bool (strict)"("DisabledEnum"=T19."Disabled and Grayed Out" ("Disabled")) -> ()  [unwired: 2 in, 2 out]
                    n2664 = case shown="True" "Start Time" {
                      selector: "Start Time" -> [_ w3211]
                      frame False {
                      }
                      frame True {
                        n2665 = Not(x=w3211) -> (.not. x?=w3210:bool)
                        n2666 = local write "Start Time"(w3210) -> ()
                        n2667 = local read "EVENT LOG"() -> (w3212:string)
                        n2668 = call "Event Log.vi"("Content"="Test in progress", "EVENT LOG"=w3212) -> ("EVENT LOG"=w3214:string)  [unwired: 8 in, 1 out]
                        n2669 = local write "EVENT LOG"(w3214) -> ()
                      }
                    }
                    n2670 = disable-structure shown="Enabled" {
                      disable-tunnel: [w3203 w3209] -> w3192
                      frame Disabled {
                        n2671 = local read "Set Hz"() -> (w3206:dbl)
                        n2672 = call <vilib>:"Uniform White Noise Waveform.vi"() -> ("signal out"=w3205:waveform(dbl))  [unwired: 10 in, 1 out]
                        n2673 = Random Number (0-1)() -> (number: 0 to 1=w3202:dbl)
                        n2674 = Add(x=w3206, y=w3205) -> (x+y=w3204:waveform(dbl))
                        n2675 = Multiply(x=ext 0.01 ("y"), y=w3202) -> (x*y=w3200:ext)
                        n2676 = Multiply(x=w3204, y=w3200) -> (x*y=w3203:waveform(ext))
                      }
                      frame Enabled {
                        n2677 = call-poly <vilib>:"Random Number (Range).vi"("lower bound (0)"=49.89, "upper bound (100)"=50.8) -> ("number"=w3209:dbl)  [unwired: 9 in]
                      }
                    }
                    "StartFlg" <- TRUE ("StartFlg")
                  }
                }
                n2678 = case shown="True" w3162 {
                  frame False {
                  }
                  frame True {
                    n2679 = local write "clk"(10.0 ("clk")) -> ()
                    n2680 = Get Date/Time In Seconds() -> (seconds since 1Jan1904=w3217:timestamp)
                    n2681 = To Double Precision Float(number=w3217) -> (double precision float=w3215:dbl)
                    n2682 = local write "acq timer"(w3215) -> ()
                    n2683 = local write "act save time"(w3215) -> ()
                  }
                }
                n2684 = call "Elapsed Time"("Time Target (s)"="Countdown", "Reset"=w3151) -> ("Elapsed Time (s)"=w3156:dbl, "Time has Elapsed"=w3154:bool)  [unwired: 10 in, 6 out]
                "Countdown 2" <- w3156
                n2685 = Subtract(x=w3156, y=2.0) -> (x-y=w3159:dbl)
                n2686 = Less?(x=w3159, y="Countdown") -> (x < y?=w3157:bool)
                n2687 = And(x=w3157, y=w3154) -> (x .and. y?=w3153:bool)
                n2688 = case shown="True" w3153 {
                  frame False {
                  }
                  frame True {
                    (unwired) dbl[] [] ("History Data")
                    n2689 = local write "Engage"(FALSE ("Engage")) -> ()
                    n2690 = local write "RUN"(TRUE ("RUN")) -> ()
                    n2691 = local read "Humidity ( %RH )"() -> (→"Rh Before":dbl)
                  }
                }
                n2692 = local read "Test \nStatus"() -> (w3149:bool)
                n2693 = Select(t=w3147, s=w3149, f=0.0) -> (s? t:f=w3148:dbl)
                n2694 = local write "Frequency ( Hz )"(w3148) -> ()
              }
              frame #1 {
                w3240 = 1000000.0 ("x")
                # "HC;1/0\nST;VALUE"
                # "Elapsed time\ncof\nstroke\nAir temp\nTemp\nHumidity"
                # "acq timer\n\nact save time"
                # "convert to microseconds"
                n2695 = local read "COUNT"() -> (w3223:i32)
                n2696 = local read "Rate"() -> (w3236:dbl)
                n2697 = Divide(x=w3240, y=w3236) -> (x/y=w3241:dbl)
                n2698 = Greater Or Equal?(x=w3223, y=250) -> (x >= y?=w3222:bool)
                n2699 = Get Date/Time In Seconds() -> (seconds since 1Jan1904=w3243:timestamp)
                n2700 = case shown="True" w3222 {
                  frame False {
                    n2701 = local read "COUNT"() -> (w3244:i32)
                    n2702 = Increment(x=w3244) -> (x+1=w3245:i32)
                    n2703 = local write "COUNT"(w3245) -> ()
                  }
                  frame True {
                    n2704 = local write "COUNT"(0 ("COUNT")) -> ()
                  }
                }
                n2705 = local read "Samplingtime 2"() -> (w3221:dbl)
                n2706 = local read "act save time"() -> (w3238:dbl)
                n2707 = Divide(x=w3241, y=w3240) -> (x/y=w3239:dbl)
                n2708 = To Double Precision Float(number=w3243) -> (double precision float=w3232:dbl)
                n2709 = Add(x=w3238, y=w3221) -> (x+y=w3237:dbl)
                n2710 = local read "acq timer"() -> (w3242:dbl)
                n2711 = local read "COUNT"() -> (w3225:i32)
                n2712 = Greater Or Equal?(x=w3232, y=w3237) -> (x >= y?=w3220:bool)
                n2713 = Multiply(x=w3239, y=w3225) -> (x*y=w3231:dbl)
                n2714 = Subtract(x=w3232, y=w3242) -> (x-y=w3234:dbl)
                n2715 = local read "Save"() -> (w3235:bool)
                n2716 = Add(x=w3234, y=w3231) -> (x+y=w3218:dbl)
                "Elapsed time 3" <- w3218
                n2717 = And(x=w3220, y=w3235) -> (x .and. y?=w3233:bool)
                n2718 = Divide(x=w3218, y=60.0) -> (x/y=w3229:dbl)
                n2719 = local read "Test \nStatus"() -> (w3219:bool)